vi "Alyssa_GlueDots.vi"() -> ()   [LabVIEW 2016]
uses:
  C:/Users/Aerotech/Documents/BNLStaveAssembly-blueprint/Bin/Aerotech.A3200.dll
  BNLStaveAssembly-blueprint/Bin/Aerotech.A3200.dll
  <vilib>/vision/Image Controls.llb/IMAQ Image.ctl
  Utils/Controls/All_Enums/Enum_TypeDef_TapeType.ctl
  <vilib>/LabVIEW Interface for Arduino/Type Defs/Arduino Resource.ctl
  <vilib>/LabVIEW Interface for Arduino/Type Defs/Board Type.ctl
  <vilib>/LabVIEW Interface for Arduino/Type Defs/Pin Mode.ctl
  <vilib>/Utility/file.llb/Read Delimited Spreadsheet (DBL).vi
  <vilib>/LabVIEW Interface for Arduino/LabVIEW Interface for Arduino.lvlib
panel:
  out "XYZ .NET Refnum out":refnum<k24>
  out "check":dbl[][](array[numeric])
  in  "?":T1(tab)
  in  "Tape Type":T2=enum."Axial (Sutcliffe NP49-01-100 01-Mar-16)"
  in  "Module corner coordinates":T3={"X [mm]"=-325.4922095457569, "Y [mm]"=111.42987050829626, "Z [mm] "=34.99996599632762}
  in  "Axis speeds (mm/s)":T4={"vX [mm]"=400.0, "vY [mm]"=400.0, "vZ [mm] "=400.0}
  in  "Home?":bool
  in  "Lowest Z Position":dbl=38.0
  out "Arduino Resource":T5={"VISA resource"="GlueCTRL", "Board Type"=enum."Uno", "Connection Type"=enum."USB / Serial", "Bytes Per Packet (15)"=15}
  in  "Digital I/O Pin":u8=7
  in  "XYZ Stage Control":refnum<k24>
  in  "Testing?":bool
  out "Difference camera/syringe in X":dbl=-133.03368290747076
  out "Difference camera/syringe in y":dbl=-2.170984960815403
  in  "um/pix resolution":dbl=1.58
  in  "Image Feed":T7=refnum
  in  "Path to save collected images":path=path "C:/Users/Aerotech/cernbox/BNL/Stave Assembly Records/2017-06-12/3"
  in  "Estimate distance y":dbl
  in  "Estimate distance x":dbl=130.0
  in  "Lowest Z position Calibration":dbl=17.0
  out "Final Position":T8={"Final X"=-325.49379764644783, "Final Y"=23.533617154160947, "Final Z"=34.99956596392527}
  out "error out":errorcluster={"status"=FALSE, "code"=1073676418, "source"="VISA Close in GlueSingleModule(SubVI).vi->2_VisualizeModulePositioning2.vi->VMP_TestStand.vi"}
  in  "error in":errorcluster
  # "Timers (ms)"
  # "Overview: This takes a pattern of zeroes/ones (.csv file) as well as the start coordinates of the top left corner of a module and places dots of glue  \nRequirements: NI Arduino dependencies\nInstructions: Select a .csv file (ones indicate regions for glue) as well as a starting coordinate (this is default to the top left corner of the module spacer). You \ncan also input axis speeds (default to maximum) and module lengths and widths (default to 90 mm) which are the widths of the module to which you want to \nplace glue. Lastly, one can choose to Home the stage here and can select the lowest position in Z. The default is that the stage moves down 2-3 mm in Z \nwhile dispensing.  The Arduino inputs are default and simply allow the LabView program to drigger the Arduino (which sends a signal to the dispenser). The \nprogram signals to dispense air- all other parameters such as length of dispensing (default: 350 millisec), pressure (default: 48 psi), and vacuum pressure \n(default: 7.8 psi) are set on the dispenser itself. The defaults are highly recommended here."
  # "Positioning Inputs"
  # "Arduino Inputs"
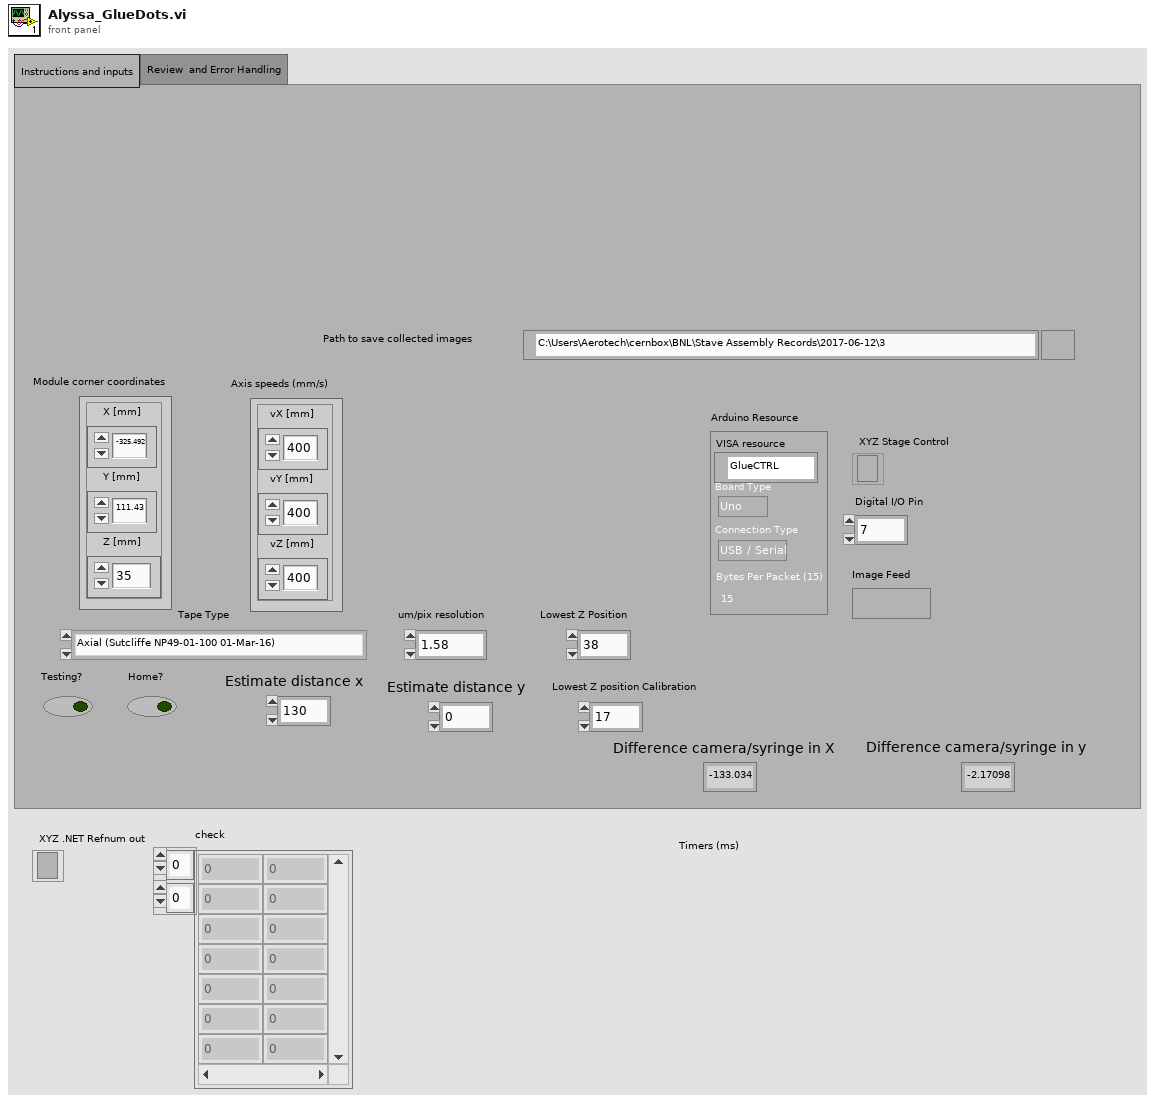
[diagram p1: front panel]
types:
  T1 = enum32{"Instructions and inputs", "Review  and Error Handling"}
  T2 = typedef "Enum_TypeDef_TapeType.ctl" = enum16{"Right stereo", "Left stereo", "Stereo (Sutcliffe NP49-01-100 01-Mar-16)", "Axial (Sutcliffe NP49-01-100 01-Mar-16)"}
  T3 = cluster{"X [mm]":dbl, "Y [mm]":dbl, "Z [mm] ":dbl}
  T4 = cluster{"vX [mm]":dbl, "vY [mm]":dbl, "vZ [mm] ":dbl}
  T5 = typedef "LabVIEW Interface for Arduino.lvlib/Arduino Resource.ctl" = cluster{"VISA resource":refnum<visa-resource-name>, "Board Type":T6, "Connection Type":enum8{"USB / Serial"}, "Bytes Per Packet (15)":u8}
  T6 = typedef "LabVIEW Interface for Arduino.lvlib/Board Type.ctl" = enum16{"Uno", "Dimuelanove w/Atmega 328", "Mega 2560"}
  T7 = typedef "IMAQ Image.ctl" = refnum<image>
  T8 = cluster{"Final X":dbl, "Final Y":dbl, "Final Z":dbl}
  T9 = typedef "LabVIEW Interface for Arduino.lvlib/Pin Mode.ctl" = enum8{"Input", "Output"}
  T10 = cluster{dbl, "Y [mm]":dbl, "Lowest Z Position":dbl}
  T11 = cluster{"Final X":dbl, "Final Y":dbl, "vZ [mm]":dbl}
  T12 = cluster{"Final X":dbl, "Final Y":dbl, "Lowest Z Position":dbl}
  T13 = cluster{"Final X":dbl, "Final Y":dbl, "Z [mm] ":dbl}
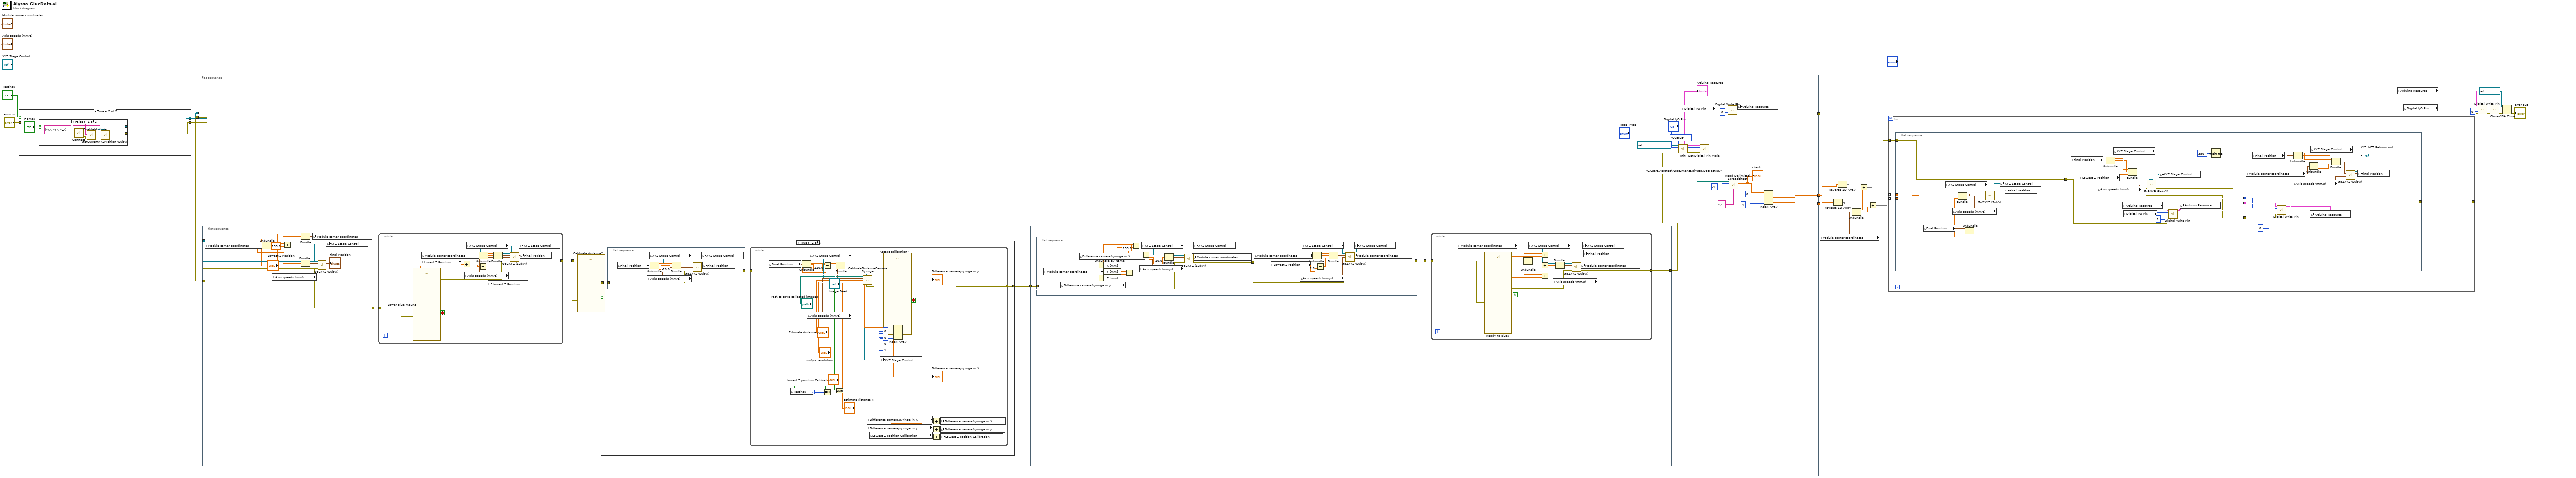
[diagram p0: block diagram]
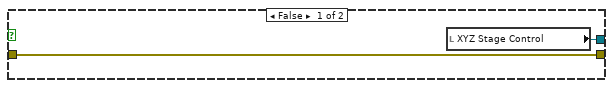
[diagram p2: hidden frame]
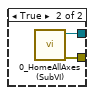
[diagram p3: hidden frame]
diagram:
  n1 = case shown="True" "Testing?" {
    tunnel: [w9 w11] -> w3
    tunnel: [w8 w10] -> w5
    tunnel: "error in" -> [w8 _]
    frame False {
      n2 = local read "XYZ Stage Control"() -> (w9:refnum<k24>)
    }
    frame True {
      n3 = case shown="False" "Home?" {
        tunnel: [w15 w21] -> w11
        tunnel: [w14 w20] -> w10
        frame False {
          w17 = string[] ["X", "Y", "Z"] ("Axes Names")
          n4 = call "Connect.vi"() -> ("error out"=w18:errorcluster, "controller"=w13:refnum<k24>)  [unwired: 10 in]
          n5 = call "EnableMultiple.vi"("error in (no error)"=w18, "axis names"=w17, "controller in"=w13) -> ("error out"=w19:errorcluster, "controller out"=w16:refnum<k24>)  [unwired: 7 in]
          n6 = call "GetCurrentXYZPosition (SubVI).vi"(".NET Refnum in - Device"=w16, "error in (no error)"=w19, "Axes Names"=w17) -> ("error out"=w14:errorcluster, ".NET Refnum out  - Device"=w15:refnum<k24>)  [unwired: 3 in, 4 out]
        }
        frame True {
          n7 = call "0_HomeAllAxes (SubVI).vi"() -> ("error out"=w20:errorcluster, "controller out"=w21:refnum<k24>)  [unwired: 8 in, 2 out]
        }
      }
    }
  }
  n8 = flat-sequence {
    tunnel: [w47] -> w7
    tunnel: w5 -> [w37]
    tunnel: w3 -> [w31]
    tunnel: [w29] -> w2
    tunnel: [w28] -> w1
    tunnel: w7 -> [w204]
    tunnel: w2 -> [w197]
    tunnel: w1 -> [w195]
    frame #0 {
      n9 = flat-sequence {
        tunnel: w37 -> [w61]
        tunnel: [w60] -> w32
        tunnel: w31 -> [w54]
        tunnel: w32 -> [w63]
        tunnel: [w62] -> w30
        tunnel: [w82] -> w34
        tunnel: w30 -> [w81]
        tunnel: w34 -> [w142]
        tunnel: [w140] -> w33
        tunnel: [w173] -> w35
        tunnel: w33 -> [w174]
        frame #0 {
          n10 = local read "Module corner coordinates"() -> (w56:T3)
          n11 = Unbundle(w56) -> ("X [mm]"=w53:dbl, "Y [mm]"=w50:dbl)  [unwired: 1 out]
          n12 = local read "Axis speeds (mm/s)"() -> (w59:T4)
          n13 = Add(x=w53, y=133.0) -> (x+y=w51:dbl)
          n14 = Bundle(w51, "Y [mm]"=w50, "Lowest Z Position"="Lowest Z Position") -> (w48:T10)  [unwired: 1 in]
          n15 = Bundle(w51, "Y [mm]"=w50, "Lowest Z Position"="Lowest Z Position") -> (w55:T10)  [unwired: 1 in]
          n16 = local write "Module corner coordinates"(w48) -> ()
          n17 = call "Go2XYZ (SubVI).vi"(".NET Refnum in"=w54, "Go to Coordinates"=w55, "Axis Speeds"=w59, "error in (no error)"=w61) -> (".NET Refnum out"=w58:refnum<k24>, "Final Position"=→"Final Position":T8, "error out"=w60:errorcluster)  [unwired: 7 in, 2 out]
          n18 = local write "XYZ Stage Control"(w58) -> ()
        }
        frame #1 {
          n19 = while {
            tunnel: w63 -> [w80]
            tunnel: [w76] -> w62
            stop <- w79 stop-if-true
            n20 = call "Lower glue mount"("error in (no error)"=w80) -> ("Move Z down"=w71:dbl, "Move Z up"=w70:dbl, "Accept current Z?"=w79:bool, "error out"=w77:errorcluster)  [unwired: 14 in, 1 out]
            n21 = local read "Lowest Z Position"() -> (w64:dbl)
            n22 = local read "Module corner coordinates"() -> (w74:T3)
            n23 = Add(x=w64, y=w71) -> (x+y=w68:dbl)
            n24 = local read "Axis speeds (mm/s)"() -> (w78:T4)
            n25 = local read "XYZ Stage Control"() -> (w66:refnum<k24>)
            n26 = Subtract(x=w68, y=w70) -> (x-y=w67:dbl)
            n27 = Unbundle(w74) -> ("X [mm]"=w73:dbl, "Y [mm]"=w72:dbl)  [unwired: 1 out]
            n28 = local write "Lowest Z Position"(w67) -> ()
            n29 = Bundle("X [mm]"=w73, "Y [mm]"=w72, w67) -> (w69:cluster{"X [mm]":dbl, "Y [mm]":dbl, dbl})  [unwired: 1 in]
            n30 = call "Go2XYZ (SubVI).vi"(".NET Refnum in"=w66, "Go to Coordinates"=w69, "Axis Speeds"=w78, "error in (no error)"=w77) -> (".NET Refnum out"=w75:refnum<k24>, "Final Position"=w65:T8, "error out"=w76:errorcluster)  [unwired: 7 in, 2 out]
            n31 = local write "XYZ Stage Control"(w75) -> ()
            n32 = local write "Final Position"(w65) -> ()
          }
        }
        frame #2 {
          n33 = call "Calibrate distance?"("error in (no error)"=w81) -> ("Calibrate distance?"=w83:bool, "error out"=w84:errorcluster)  [unwired: 16 in, 1 out]
          n34 = case shown="True" w83 {
            tunnel: w84 -> [w85 w87]
            tunnel: [w85 w88] -> w82
            frame False {
            }
            frame True {
              n35 = flat-sequence {
                tunnel: w87 -> [w90]
                tunnel: [w89] -> w86
                frame #0 {
                  n36 = local read "Final Position"() -> (w97:T8)
                  n37 = local read "Axis speeds (mm/s)"() -> (w93:T4)
                  n38 = local read "XYZ Stage Control"() -> (w92:refnum<k24>)
                  n39 = Unbundle(w97) -> ("Final X"=w95:dbl, "Final Y"=w96:dbl)  [unwired: 1 out]
                  n40 = Bundle("Final X"=w95, "Final Y"=w96, "vZ [mm]"=-20.0) -> (w99:T11)  [unwired: 1 in]
                  n41 = call "Go2XYZ (SubVI).vi"(".NET Refnum in"=w92, "Go to Coordinates"=w99, "Axis Speeds"=w93, "error in (no error)"=w90) -> (".NET Refnum out"=w91:refnum<k24>, "Final Position"=w94:T8, "error out"=w89:errorcluster)  [unwired: 7 in, 2 out]
                  n42 = local write "XYZ Stage Control"(w91) -> ()
                  n43 = local write "Final Position"(w94) -> ()
                }
              }
              n44 = while {
                tunnel: [w138] -> w88
                tunnel: w86 -> [w126]
                i -> [w123]
                stop <- w139 stop-if-true
                n45 = local read "Final Position"() -> (w100:T8)
                n46 = local read "Testing?"() -> (w121:bool)
                n47 = Unbundle(w100) -> ("Final X"=w105:dbl, "Final Y"=w103:dbl, "Final Z"=w104:dbl)
                n48 = local read "Axis speeds (mm/s)"() -> (w128:T4)
                n49 = local read "XYZ Stage Control"() -> (w124:refnum<k24>)
                n50 = Equal To 0?(x=w123) -> (x = 0?=w122:bool)
                n51 = Subtract(x=w103, y=220.0) -> (x-y=w101:dbl)
                n52 = And(x=w121, y=w122) -> (x .and. y?=w120:bool)
                n53 = Bundle("Final X"=w105, w101, "Final Z"=w104) -> (w106:cluster{"Final X":dbl, dbl, "Final Z":dbl})  [unwired: 1 in]
                n54 = call "CalibrateDistanceCameraSyringe.vi"("Path to save collected images"="Path to save collected images", "Image Feed"="Image Feed", "Off stave position"=w106, ".NET Refnum in"=w124, "Axis speeds (mm/s)"=w128, "Lowest Z Position"="Lowest Z position Calibration", "Estimate distance y"="Estimate distance y", "um/pix resolution"="um/pix resolution", "Estimate distance x"="Estimate distance x", "error in"=w126, "Testing?"=w120) -> ("XYZ .NET Refnum out"=w127:refnum<k24>, "error out"=w125:errorcluster, "X/Y difference (CAMERA - SYRINGE)"=w135:dbl[][])  [unwired: 2 in]
                n55 = local read "Difference camera/syringe in X"() -> (w110:dbl)
                n56 = local read "Difference camera/syringe in y"() -> (w107:dbl)
                n57 = local read "Lowest Z position Calibration"() -> (w112:dbl)
                n58 = local write "XYZ Stage Control"(w127) -> ()
                n59 = call "Accept calibration?"("error in (no error)"=w125) -> ("Change in lowest Z"=w114:dbl, "Change in distance Y estimate"=w115:dbl, "Change in distance X estimate"=w116:dbl, "Accept the distance syringe/camera?"=w139:bool, "error out"=w138:errorcluster)  [unwired: 13 in, 1 out]
                n60 = Index Array(array=w135, index (row) #1=0 ("index (row)"), index (col) #1=0 ("disabled index (col)"), index (row) #2=0 ("index (row)"), index (col) #2=1 ("disabled index (col)")) -> (element #1=→"Difference camera/syringe in X":dbl, element #2=→"Difference camera/syringe in y":dbl)
                n61 = Add(x=w110, y=w116) -> (x+y=w109:dbl)
                n62 = Add(x=w107, y=w115) -> (x+y=w108:dbl)
                n63 = Add(x=w112, y=w114) -> (x+y=w113:dbl)
                n64 = local write "Difference camera/syringe in X"(w109) -> ()
                n65 = local write "Difference camera/syringe in y"(w108) -> ()
                n66 = local write "Lowest Z position Calibration"(w113) -> ()
              }
            }
          }
        }
        frame #3 {
          n67 = flat-sequence {
            tunnel: w142 -> [w149]
            tunnel: [w146] -> w141
            tunnel: [w160] -> w140
            tunnel: w141 -> [w161]
            frame #0 {
              n68 = local read "Module corner coordinates"() -> (w159:T3)
              n69 = local read "Difference camera/syringe in y"() -> (w154:dbl)
              n70 = local read "Difference camera/syringe in X"() -> (w155:dbl)
              n71 = Unbundle By Name(w159) -> ("X [mm]"=w145:dbl, "Y [mm]"=w158:dbl)  [unwired: 1 out]
              n72 = Subtract(x=w158, y=w154) -> (x-y=w156:dbl)
              n73 = Subtract(x=w145, y=133.0) -> (x-y=w143:dbl)
              n74 = local read "Axis speeds (mm/s)"() -> (w150:T4)
              n75 = local read "XYZ Stage Control"() -> (w151:refnum<k24>)
              n76 = Subtract(x=w143, y=w155) -> (x-y=w157:dbl)
              n77 = Bundle(w157, w156, "index (row)"=-20.0) -> (w148:cluster{dbl, dbl, "index (row)":dbl})  [unwired: 1 in]
              n78 = call "Go2XYZ (SubVI).vi"(".NET Refnum in"=w151, "Go to Coordinates"=w148, "Axis Speeds"=w150, "error in (no error)"=w149) -> (".NET Refnum out"=w152:refnum<k24>, "Final Position"=w153:T8, "error out"=w146:errorcluster)  [unwired: 7 in, 2 out]
              n79 = local write "Module corner coordinates"(w153) -> ()
              n80 = local write "XYZ Stage Control"(w152) -> ()
            }
            frame #1 {
              n81 = local read "Module corner coordinates"() -> (w166:T3)
              n82 = local read "Lowest Z Position"() -> (w169:dbl)
              n83 = local read "Axis speeds (mm/s)"() -> (w163:T4)
              n84 = local read "XYZ Stage Control"() -> (w162:refnum<k24>)
              n85 = Unbundle(w166) -> ("X [mm]"=w167:dbl, "Y [mm]"=w168:dbl)  [unwired: 1 out]
              n86 = Subtract(x=w169, y=2.0) -> (x-y=w171:dbl)
              n87 = Bundle("X [mm]"=w167, "Y [mm]"=w168, w171) -> (w172:cluster{"X [mm]":dbl, "Y [mm]":dbl, dbl})  [unwired: 1 in]
              n88 = call "Go2XYZ (SubVI).vi"(".NET Refnum in"=w162, "Go to Coordinates"=w172, "Axis Speeds"=w163, "error in (no error)"=w161) -> (".NET Refnum out"=w164:refnum<k24>, "Final Position"=w165:T8, "error out"=w160:errorcluster)  [unwired: 7 in, 2 out]
              n89 = local write "Module corner coordinates"(w165) -> ()
              n90 = local write "XYZ Stage Control"(w164) -> ()
            }
          }
        }
        frame #4 {
          n91 = while {
            tunnel: w174 -> [w188]
            tunnel: [w190] -> w173
            stop <- w175 continue-if-true
            n92 = local read "Module corner coordinates"() -> (w187:T3)
            n93 = call "Ready to glue?"("error in (no error)"=w188) -> ("Move in Z"=w184:dbl, "Move in Y"=w185:dbl, "Move in X"=w186:dbl, "Oh yeah! Reset Arduino and go!"=w175:bool, "error out"=w189:errorcluster)  [unwired: 13 in, 1 out]
            n94 = Unbundle(w187) -> ("X [mm]"=w183:dbl, "Y [mm]"=w182:dbl, "Z [mm]"=w181:dbl)
            n95 = local read "XYZ Stage Control"() -> (w191:refnum<k24>)
            n96 = Add(x=w183, y=w186) -> (x+y=w178:dbl)
            n97 = Add(x=w182, y=w185) -> (x+y=w180:dbl)
            n98 = Add(x=w181, y=w184) -> (x+y=w179:dbl)
            n99 = local read "Axis speeds (mm/s)"() -> (w193:T4)
            n100 = Bundle(w178, w180, w179) -> (w177:cluster{dbl, dbl, dbl})  [unwired: 1 in]
            n101 = call "Go2XYZ (SubVI).vi"(".NET Refnum in"=w191, "Go to Coordinates"=w177, "Axis Speeds"=w193, "error in (no error)"=w189) -> (".NET Refnum out"=w192:refnum<k24>, "Final Position"=w176:T8, "error out"=w190:errorcluster)  [unwired: 7 in, 2 out]
            n102 = local write "Module corner coordinates"(w176) -> ()
            n103 = local write "XYZ Stage Control"(w192) -> ()
            n104 = local write "Final Position"(w176) -> ()
          }
        }
      }
      n105 = call <vilib>:"Init.vi"("VISA resource"=refnum<visa-resource-name> "GlueCTRL", "error in"=w35) -> ("Arduino Resource"=w39:T5, "error out"=w40:errorcluster)  [unwired: 16 in]
      "Arduino Resource" <- w39
      n106 = local read "Digital I/O Pin"() -> (w36:u8)
      n107 = call <vilib>:"Set Digital Pin Mode.vi"("Arduino Resource"=w39, "Digital I/O Pin"="Digital I/O Pin", "Pin Mode (Input)"=Pin_Mode."Output", "error in"=w40) -> ("Arduino Resource"=w43:T5, "error out"=w44:errorcluster)  [unwired: 10 in]
      n108 = call <vilib>:"Digital Write Pin.vi"("Arduino Resource"=w43, "Digital I/O Pin (0)"=w36, "Value (0)"=u8 0, "error in"=w44) -> ("Arduino Resource"=w38:T5, "error out"=w47:errorcluster)  [unwired: 10 in]
      n109 = call-poly <vilib>:"Read Delimited Spreadsheet.vi"("file path (dialog if empty)"=path "C:/Users/Aerotech/Documents/alyssa/DotTest.csv", "number of rows (all:-1)"=-1, "delimiter (\\t)"="," ("delimiter (\\t)")) -> ("all rows"=w24:dbl[][])  [unwired: 7 in, 5 out]
      "check" <- w24
      n110 = local write "Arduino Resource"(w38) -> ()
      n111 = Index Array(array=w24, index (col) #1=0 ("index"), index (col) #2=1 ("index")) -> (element #1=w29:dbl[], element #2=w28:dbl[])  [unwired: 2 in]
    }
    frame #1 {
      n112 = local read "Module corner coordinates"() -> (w202:T3)
      n113 = Reverse 1D Array(array=w195) -> (reversed array=w194:dbl[])
      n114 = Reverse 1D Array(array=w197) -> (reversed array=w196:dbl[])
      n115 = Unbundle(w202) -> ("X [mm]"=w198:dbl, "Y [mm]"=w201:dbl)  [unwired: 1 out]
      n116 = Add(x=w196, y=w198) -> (x+y=w199:dbl[])
      n117 = Add(x=w194, y=w201) -> (x+y=w200:dbl[])
      n118 = for {
        tunnel: w199 -> [w218] mode=indexing
        tunnel: w200 -> [w217] mode=indexing
        tunnel: w204 -> [w216]
        tunnel: [w214] -> w203
        n119 = flat-sequence {
          tunnel: [w230] -> w213
          tunnel: w218 -> [w229]
          tunnel: w217 -> [w228]
          tunnel: w216 -> [w230]
          tunnel: [w236] -> w220
          tunnel: [w235] -> w219
          tunnel: w213 -> [w234]
          tunnel: [w232] -> w215
          tunnel: [w262] -> w214
          tunnel: w215 -> [w247]
          tunnel: w219 -> [w261]
          tunnel: w220 -> [w259]
          frame #0 {
            n120 = local read "Final Position"() -> (w222:T8)
            n121 = local read "XYZ Stage Control"() -> (w225:refnum<k24>)
            n122 = local read "Axis speeds (mm/s)"() -> (w226:T4)
            n123 = Unbundle(w222) -> ("Final Z"=w221:dbl)  [unwired: 2 out]
            n124 = Bundle(w229, w228, "Final Z"=w221) -> (w227:cluster{dbl, dbl, "Final Z":dbl})  [unwired: 1 in]
            n125 = call "Go2XYZ (SubVI).vi"(".NET Refnum in"=w225, "Go to Coordinates"=w227, "Axis Speeds"=w226) -> (".NET Refnum out"=w223:refnum<k24>, "Final Position"=w224:T8)  [unwired: 8 in, 3 out]
            n126 = local write "XYZ Stage Control"(w223) -> ()
            n127 = local write "Final Position"(w224) -> ()
          }
          frame #1 {
            n128 = local read "Final Position"() -> (w246:T8)
            n129 = local read "Lowest Z Position"() -> (w243:dbl)
            n130 = local read "Axis speeds (mm/s)"() -> (w241:T4)
            n131 = Unbundle(w246) -> ("Final X"=w245:dbl, "Final Y"=w244:dbl)  [unwired: 1 out]
            n132 = local read "XYZ Stage Control"() -> (w240:refnum<k24>)
            n133 = local read "Arduino Resource"() -> (w237:T5)
            n134 = local read "Digital I/O Pin"() -> (w236:u8)
            n135 = Bundle("Final X"=w245, "Final Y"=w244, "Lowest Z Position"=w243) -> (w242:T12)  [unwired: 1 in]
            n136 = call <vilib>:"Digital Write Pin.vi"("Arduino Resource"=w237, "Digital I/O Pin (0)"=w236, "Value (0)"=u8 1, "error in"=w234) -> ("Arduino Resource"=w235:T5, "error out"=w233:errorcluster)  [unwired: 10 in]
            n137 = call "Go2XYZ (SubVI).vi"(".NET Refnum in"=w240, "Go to Coordinates"=w242, "Axis Speeds"=w241, "error in (no error)"=w233) -> (".NET Refnum out"=w239:refnum<k24>, "error out"=w232:errorcluster)  [unwired: 7 in, 3 out]
            n138 = local write "XYZ Stage Control"(w239) -> ()
            n139 = local write "Arduino Resource"(w235) -> ()
            n140 = Wait (ms)(milliseconds to wait=u32 350) -> ()  [unwired: 1 out]
          }
          frame #2 {
            n141 = local read "Module corner coordinates"() -> (w256:T3)
            n142 = local read "Final Position"() -> (w257:T8)
            n143 = call <vilib>:"Digital Write Pin.vi"("Arduino Resource"=w261, "Digital I/O Pin (0)"=w259, "Value (0)"=u8 0, "error in"=w247) -> ("Arduino Resource"=w258:T5, "error out"=w262:errorcluster)  [unwired: 10 in]
            n144 = local read "Axis speeds (mm/s)"() -> (w251:T4)
            n145 = Unbundle(w257) -> ("Final X"=w255:dbl, "Final Y"=w254:dbl)  [unwired: 1 out]
            n146 = Unbundle(w256) -> ("Z [mm]"=w253:dbl)  [unwired: 2 out]
            n147 = local write "Arduino Resource"(w258) -> ()
            n148 = local read "XYZ Stage Control"() -> (w250:refnum<k24>)
            n149 = Bundle("Final X"=w255, "Final Y"=w254, "Z [mm]"=w253) -> (w252:T13)  [unwired: 1 in]
            n150 = call "Go2XYZ (SubVI).vi"(".NET Refnum in"=w250, "Go to Coordinates"=w252, "Axis Speeds"=w251) -> (".NET Refnum out"=→"XYZ .NET Refnum out":refnum<k24>, "Final Position"=w249:T8)  [unwired: 8 in, 3 out]
            n151 = local write "Final Position"(w249) -> ()
          }
        }
      }
      n152 = local read "Arduino Resource"() -> (w210:T5)
      n153 = local read "Digital I/O Pin"() -> (w211:u8)
      n154 = call <vilib>:"Digital Write Pin.vi"("Arduino Resource"=w210, "Digital I/O Pin (0)"=w211, "Value (0)"=u8 0, "error in"=w203) -> ("Arduino Resource"=w208:T5, "error out"=w207:errorcluster)  [unwired: 10 in]
      n155 = call <vilib>:"Close.vi"("Arduino Resource"=w208, "error in"=w207) -> ("error out"=w206:errorcluster)  [unwired: 13 in]
      n156 = VISA Close(VISA resource name=refnum<visa-resource-name> "COM3", error in (no error)=w206) -> (error out=→"error out":errorcluster)
    }
  }
